vi "UHR-Fleezers Control (host) - 10.8MV_trial2.vi"() -> ()   [LabVIEW 2010] (continued)
        n697 = xnode "Read/Write Control"("FPGA VI Reference In"=w3157, "error in"=w3156, "Invert APD Gate"=w3154, "APD Gate ON Count"=w3153, "APD Gate OFF Count"=w3152, "APD Acq Rate Count"=w3148, "APD Gate Operating Mode"=w3151, "APD 1 AO scale factor"=w3146, "APD 2 AO scale factor"=w3145) -> ("error out"=w3155:errorcluster)  [unwired: 1 out]
      }
      event "GI Frequency, ON count", "Green FB Count", "GI Frequency, OFF count": Value Change {
        n698 = event-data() -> ()  [unwired: 7 out]
        n699 = xnode "Read/Write Control"("FPGA VI Reference In"=w3321, "error in"=w3319, "Green interlace ON count"="GI Frequency, ON count", "Green interlace OFF count"="GI Frequency, OFF count", "Green interlace ON count 2"="GI Frequency, ON count", "Green interlace OFF count 2"="GI Frequency, OFF count", "Green FB Count"="Green FB Count") -> ("error out"=w3320:errorcluster)  [unwired: 1 out]
      }
      event "Number of F/B Scans (AOD)", "Scan Speed (nm/s)", "Scan BD", "Initial delta (MHz)", "Step Size (nm)", "Scan Range (nm)": Value Change {
        w3500 = 123.0  # AOM cal (nm/MHz)
        n700 = event-data() -> ()  [unwired: 7 out]
        n701 = local read "BD 1 Frequency 1 (MHz)"() -> (w3483:dbl)
        n702 = local read "AOM X Cal (nm/MHz)"() -> (w3475:dbl)
        n703 = local read "X RF Frequency Limits (MHz)"() -> (w3487:T16)
        n704 = local read "Y RF Frequency Limits (MHz)"() -> (w3484:T16)
        n705 = local read "BD 2 Frequency 1 (MHz)"() -> (w3489:dbl)
        n706 = Negate(x="Scan Range (nm)") -> (-x=w3453:dbl)
        n707 = Divide(x=w3453, y=w3475) -> (x/y=w3457:dbl)
        n708 = Select(t=w3487, s="Scan BD", f=w3484) -> (s? t:f=w3486:T16)
        n709 = Select(t=w3483, s="Scan BD", f=w3489) -> (s? t:f=w3488:dbl)
        n710 = Unbundle By Name(w3486) -> ("Maximum"=w3495:dbl, "Minimum"=w3494:dbl)
        n711 = Add(x=w3457, y=w3488) -> (x+y=w3492:dbl)
        n712 = Divide(x=w3453, y="Step Size (nm)") -> (x/y=w3472:dbl)
        n713 = Divide(x="Step Size (nm)", y=w3475) -> (x/y=w3481:dbl)
        n714 = Absolute Value(x=w3472) -> (abs(x)=w3456:dbl)
        n715 = Sign(1:w3453) -> (0:w3454:dbl)
        n716 = In Range and Coerce(upper limit=w3495, x=w3492, lower limit=w3494) -> (coerced(x)=w3491:dbl, In Range?=w3493:bool)
        n717 = To Unsigned Quad Integer(1:w3456) -> (0:w3471:u64)
        "Scan steps (AOD)" <- w3471
        n718 = call "IR AOM freq to word.vi"("Frequency In (MHz)"=w3481) -> ("Frequency Word Out (double)"=w3478:dbl)
        n719 = Multiply(x=w3454, y=w3478) -> (x*y=w3455:dbl)
        n720 = Subtract(x=w3492, y=w3491) -> (x-y=w3490:dbl)
        n721 = To Quad Integer(1:w3455) -> (0:w3477:i64)
        "Incr. int (AOD)" <- w3477
        n722 = Subtract(x=w3457, y=w3490) -> (x-y=w3476:dbl)
        "Scan Range (MHz)" <- w3476
        n723 = Select(t=w3457, s=w3493, f=w3476) -> (s? t:f=w3496:dbl)
        n724 = Multiply(x=w3476, y=w3475) -> (x*y=w3474:dbl)
        n725 = Decrement(x=w3471) -> (x-1=w3524:u64)
        n726 = Negate(x=w3474) -> (-x=w3470:dbl)
        n727 = local write "Scan Range (nm)"(w3470) -> ()
        n728 = Divide(x=w3496, y=w3524) -> (x/y=w3480:dbl)
        "Scan Increment (MHz)" <- w3480
        n729 = call "IR AOM freq to word.vi"("Frequency In (MHz)"=w3480) -> ("Frequency Word Out (double)"=w3479:dbl)
        n730 = Divide(x="Step Size (nm)", y="Scan Speed (nm/s)") -> (x/y=w3467:dbl)
        n731 = To Quad Integer(1:w3479) -> ()  [unwired: 1 out]
        n732 = local read "Number Interlace Sets"() -> (w3451:u8)
        n733 = local read "AI Count (ticks)"() -> (w3452:u32)
        n734 = local read "Total Counts (ticks)"() -> (w3450:u32)
        n735 = local read "# Samples/trap"() -> (w3482:u32)
        n736 = Multiply(x=w3452, y=w3451) -> (x*y=w3449:u32)
        n737 = Divide(x=w3450, y=w3449) -> (x/y=w3448:dbl)
        n738 = Select(t=w3483, s="Scan BD", f=w3489) -> (s? t:f=w3521:dbl)
        "Initial freq. (MHz)" <- w3521
        n739 = Add(x=w3496, y=w3521) -> (x+y=→"Final freq. (MHz)":dbl)
        n740 = Divide(x=w3450, y=40000000.0) -> (x/y=w3466:dbl)
        n741 = Divide(x=w3467, y=w3466) -> (x/y=w3465:dbl)
        n742 = To Unsigned Quad Integer(1:w3465) -> (0:w3440:u64)
        n743 = Quotient & Remainder(x=w3440, y=u64 2) -> (x-y*floor(x/y)=w3444:u64)  [unwired: 1 out]
        n744 = Equal?(x=w3444, y=u64 0) -> (x = y?=w3442:bool)
        n745 = Decrement(x=w3440) -> (x-1=w3441:u64)
        n746 = Select(t=w3440, s=w3442, f=w3441) -> (s? t:f=w3439:u64)
        "Cycles/step (AOD)" <- w3439
        n747 = xnode "Read/Write Control"("FPGA VI Reference In"=w3532, "error in"=w3531, "Scan steps"=w3471, "Number of scans"="Number of F/B Scans (AOD)", "Cycles per step"=w3439, "Scan freq.  increment"=w3477, "Scan BD"="Scan BD") -> ("error out"=w3530:errorcluster)  [unwired: 1 out]
        n748 = Multiply(x=w3471, y=w3439) -> (x*y=w3525:u64)
        n749 = Multiply(x=w3525, y=u64 2) -> (x*y=w3447:u64)
        n750 = Multiply(x=w3448, y=w3447) -> (x*y=w3446:dbl)
        "Data points/scan (f/b)" <- w3446
        n751 = Multiply(x=w3446, y="Number of F/B Scans (AOD)") -> (x*y=w3528:dbl)
        "Data points/scans" <- w3528
        n752 = Divide(x=w3528, y=w3482) -> (x/y=→"N sets should be saved":dbl)
        n753 = Multiply(x=w3525, y=w3466) -> (x*y=w3464:dbl)
        "Time/Scan (s) (AOD)" <- w3464
        n754 = Select(t=w3496, s="Scan BD", f=0.0) -> (s? t:f=w3522:dbl)
        n755 = Select(t=0.0, s="Scan BD", f=w3496) -> (s? t:f=w3518:dbl)
        n756 = local read "BD 2 Frequency 2 (MHz)"() -> (w3514:dbl)
        n757 = local read "BD 1 Frequency 2 (MHz)"() -> (w3517:dbl)
        n758 = Add(x=w3518, y=w3489) -> (x+y=w3515:dbl)
        n759 = Add(x=w3483, y=w3522) -> (x+y=w3516:dbl)
        n760 = Multiply(x=w3464, y=2.0) -> (x*y=w3463:dbl)
        n761 = Multiply(x=w3463, y="Number of F/B Scans (AOD)") -> (x*y=w3460:dbl)
        n762 = Divide(x=w3460, y=60.0) -> (x/y=→"Time to Finish All (min)":dbl)
        n763 = Add(x="Trap 2 Bead Size (nm)", y="Trap 1 Bead Size (nm)") -> (x+y=w3504:dbl)
        n764 = local read "Initial delta (MHz)"() -> (w3501:dbl)
        n765 = Divide(x=w3504, y=2.0) -> (x/y=w3498:dbl)
        n766 = Subtract(x=w3515, y=w3514) -> (x-y=w3512:dbl)
        n767 = Subtract(x=w3516, y=w3517) -> (x-y=w3513:dbl)
        n768 = Square(x=w3512) -> (x^2=w3511:dbl)
        n769 = Square(x=w3513) -> (x^2=w3510:dbl)
        n770 = Add(x=w3510, y=w3511) -> (x+y=w3509:dbl)
        n771 = Square Root(x=w3509) -> (sqrt(x)=w3508:dbl)
        "Final delta (MHz)" <- w3508
        n772 = Multiply(x=w3500, y=w3508) -> (x*y=w3507:dbl)
        n773 = Multiply(x=w3501, y=w3500) -> (x*y=w3499:dbl)
        n774 = Subtract(x=w3499, y=w3498) -> (x-y=→"Initial sep (nm)":dbl)
        n775 = Subtract(x=w3507, y=w3498) -> (x-y=→"Final sep (nm)":dbl)
      }
      event "Raster Scanning...": Value Change {
        n776 = event-data() -> ("NewVal"=w3669:bool)  [unwired: 6 out]
        n777 = case shown="True" w3669 {
          frame False {
          }
          frame True {
            n778 = property on="BD 1 Frequency 1 (MHz)" class="DigNum (strict)"("Val(Sgnl)"=65.0 ("Value (Signaling)")) -> ()  [unwired: 2 in, 2 out]
          }
        }
      }
      event "Freq or Amp switch first", "Swap F1 and F2", "Freq switch delay", "Amp switch delay": Value Change {
        n779 = event-data() -> ()  [unwired: 7 out]
        n780 = local read "Freq or Amp switch first"() -> (w3671:bool)
        n781 = local read "Amp switch delay"() -> (w3672:u16)
        n782 = local read "Freq switch delay"() -> (w3674:u16)
        n783 = local read "Swap F1 and F2"() -> (w3673:bool)
        n784 = xnode "Read/Write Control"("FPGA VI Reference In"=w3677, "error in"=w3676, "Freq switch delay"=w3674, "Swap F1 and F2"=w3673, "Amp switch delay"=w3672, "Freq or Amp switch first"=w3671) -> ("error out"=w3675:errorcluster)  [unwired: 1 out]
      }
      event "Scan steps (MCL)", "Number of scans (MCL)", "Scan Range (V)\n(of steps)", "2D or 1D Scan", "N APD Samp/step", "Fast Scan Dir", "Continuous MCL Scanning", "Scan lines (y)": Value Change {
        w3778 = 32767.0 ("y")
        n785 = event-data() -> ()  [unwired: 7 out]
        n786 = Select(t="Scan lines (y)", s="2D or 1D Scan", f="Number of scans (MCL)") -> (s? t:f=w3783:u64)
        n787 = Decrement(x="Scan steps (MCL)") -> (x-1=w3799:u64)
        n788 = Divide(x="Scan Range (V)\n(of steps)", y=w3799) -> (x/y=w3798:dbl)
        "Desired Scan Incr (V)" <- w3798
        n789 = local read "APD Integration Time (s)"() -> (w3791:dbl)
        n790 = Multiply(x=w3798, y=w3778) -> (x*y=w3807:dbl)
        n791 = Divide(x=w3807, y=10.0) -> (x/y=w3797:dbl)
        "Desired incr (int)" <- w3797
        n792 = local read "Update Count (MCL)"() -> (w3803:u32)
        n793 = Round Toward -Infinity(1:w3797) -> (0:w3806:dbl)
        n794 = To Word Integer(number=w3806) -> (16bit integer=w3781:i16)
        "Actual Incr. int (MCL)" <- w3781
        n795 = Multiply(x=w3791, y=40000000.0) -> (x*y=w3804:dbl)
        n796 = Divide(x=w3804, y=w3803) -> (x/y=w3802:dbl)
        n797 = Multiply(x=i16 10, y=w3781) -> (x*y=w3779:i16)
        n798 = Multiply(x="N APD Samp/step", y=w3802) -> (x*y=w3801:dbl)
        "Cycles/step (MCL)" <- w3801
        n799 = Divide(x=w3779, y=w3778) -> (x/y=→"Actual MCL Inc (V)":dbl)
        n800 = Multiply(x="N APD Samp/step", y="Scan steps (MCL)") -> (x*y=w3793:dbl)
        n801 = local read "APD Samples/FIFO Acq."() -> (w3790:dbl)
        n802 = Multiply(x=w3793, y=u64 2) -> (x*y=w3792:dbl)
        "Data points/scan (f+b)" <- w3792
        n803 = Multiply(x=w3792, y=w3783) -> (x*y=w3810:dbl)
        "Data points/scans (MCL)" <- w3810
        n804 = Multiply(x=w3791, y=w3792) -> (x*y=w3784:dbl)
        "Time/f+b scan (s) (MCL)" <- w3784
        n805 = Divide(x=w3810, y=w3790) -> (x/y=→"N sets should be saved (MCL)":dbl)
        n806 = Multiply(x=w3784, y=w3783) -> (x*y=→"Total Time (s)":dbl)
        n807 = Not(x="Fast Scan Dir") -> (.not. x?=w3788:bool)
        n808 = xnode "Read/Write Control"("FPGA VI Reference In"=w3814, "error in"=w3813, "Scan steps (MCL)"="Scan steps (MCL)", "Number of scans (MCL)"=w3783, "Cycles per step (MCL)"=w3801, "Scan freq.  increment (MCL)"=w3781, "1D or 2D Scan?"="2D or 1D Scan", "MCL Scan Axis"=w3788, "Cont. Scan (MCL)"="Continuous MCL Scanning") -> ("error out"=w3812:errorcluster)  [unwired: 1 out]
      }
      event "Read Cal": Value Change {
        w3988 = 1000.0 ("y")
        n809 = event-data() -> ()  [unwired: 7 out]
        n810 = local read "Save file name"() -> (w4013:path)
        n811 = local write "Read Cal"(FALSE ("Read Cal")) -> ()
        n812 = Strip Path(path=w4013) -> (stripped path=w4012:path)  [unwired: 1 out]
        n813 = Path To String(path=w4012) -> (string=w4011:string)
        n814 = Concatenate Strings(w4011, "\\current.cal" ("string")) -> (w4009:string)
        n815 = String To Path(string=w4009) -> (path=w4008:path)
        n816 = Open/Create/Replace File(file path (use dialog)=w4008, operation (0:open)=T25."open", access (0:read/write)=enum16{"read/write", "read-only", "write-only"}."read-only") -> (refnum out=w4016:refnum<file>, error out=w4002:errorcluster)  [unwired: 1 in, 3 out]
        n817 = Deny Access(4:w4002, 7:w4016) -> (0:w4001:errorcluster, 3:w4007:refnum<file>)  [unwired: 1 out]
        n818 = Read from Binary File(5:0.0, 8:w4001, 9:T31."big-endian, network order" ("byte order (0:big-endian, network order)"), 10:-1 ("count (1)"), 11:w4007) -> (0:w4000:errorcluster, 2:w3998:dbl[], 3:w4003:refnum<file>)  [unwired: 2 out]
        n819 = Array To Cluster(array=w3998) -> (cluster=w3997:T33)
        n820 = Unbundle(w3997) -> ("[0]"=w3996:dbl, "[1]"=w3995:dbl, "[2]"=w3994:dbl, "[3]"=w3993:dbl, "[4]"=w3992:dbl, "[5]"=w3991:dbl)
        n821 = Close File(refnum=w4003, error in=w4000) -> (error out=→"Read cal error":errorcluster)  [unwired: 1 out]
        n822 = Multiply(x=w3991, y=w3988) -> (x*y=w3989:dbl)
        n823 = local write "T2 kappa_x (pN/nm)"(w3993) -> ()
        n824 = local write "T1 kappa_x (pN/nm)"(w3994) -> ()
        n825 = local write "T1 alpha_x (nm/V)"(w3996) -> ()
        n826 = local write "T2 alpha_x (nm/V)"(w3995) -> ()
        n827 = Multiply(x=w3992, y=w3988) -> (x*y=w3990:dbl)
        n828 = local write "T1 offset_x (mV)"(w3990) -> ()
        n829 = local write "T2 offset_x (mV)"(w3989) -> ()
      }
      event "Abort MCL Scan": Value Change {
        n830 = event-data() -> ()  [unwired: 7 out]
        n831 = local write "MCL Scanning"(FALSE ("MCL Scanning")) -> ()
        n832 = xnode "Read/Write Control"("FPGA VI Reference In"=w4021, "error in"=w4020, "Abort scan (MCL)"="Abort MCL Scan") -> ("error out"=w4019:errorcluster)  [unwired: 1 out]
      }
      event "Update Count (MCL)": Value Change {
        n833 = event-data() -> ()  [unwired: 7 out]
        n834 = xnode "Read/Write Control"("FPGA VI Reference In"=w4063, "error in"=w4062, "MCL count"="Update Count (MCL)") -> ("error out"=w4061:errorcluster)  [unwired: 1 out]
      }
      event "Phase adjust (MCL)", "+ phase (MCL)", "- phase (MCL)": Value Change {
        n835 = event-data() -> ()  [unwired: 7 out]
        n836 = Negate(x="Phase adjust (MCL)") -> (-x=w4109:i16)
        n837 = Select(t=w4109, s="- phase (MCL)", f="Phase adjust (MCL)") -> (s? t:f=w4107:i16)
        n838 = Or(x="- phase (MCL)", y="+ phase (MCL)") -> (x .or. y?=w4102:bool)
        n839 = xnode "Read/Write Control"("FPGA VI Reference In"=w4111, "error in"=w4110, "Phase count adjustment (MCL)"=w4107) -> ("FPGA VI Reference Out"=w4103:T19, "error out"=w4104:errorcluster)
        n840 = xnode "Read/Write Control"("FPGA VI Reference In"=w4103, "error in"=w4104, "+ phase (MCL)"=w4102) -> ("error out"=w4101:errorcluster)  [unwired: 1 out]
      }
      event "Abort AOD Scan": Value Change {
        n841 = event-data() -> ()  [unwired: 7 out]
        n842 = xnode "Read/Write Control"("FPGA VI Reference In"=w4190, "error in"=w4189, "Abort scan"="Abort AOD Scan") -> ("error out"=w4188:errorcluster)  [unwired: 1 out]
      }
      event "Continuous AOD Scanning": Value Change {
        n843 = event-data() -> ()  [unwired: 7 out]
        n844 = xnode "Read/Write Control"("FPGA VI Reference In"=w4232, "error in"=w4231, "Cont. Scan"="Continuous AOD Scanning") -> ("error out"=w4230:errorcluster)  [unwired: 1 out]
      }
      event "Index": Value Change {
        n845 = event-data() -> ()  [unwired: 7 out]
        n846 = call "Create new save file.vi"("Insert"="", "Ext"=".dat" ("string"), "Index In"="Index") -> ("Path Out"=→"Save file name":path, "Index Out"=w4271:dbl)
        "Save index" <- w4271
        n847 = local write "Index"(w4271) -> ()
      }
      event "AO1", "AO2": Value Change {
        w4286 = 10.0 ("y")
        w4285 = 32767.0 ("y")
        n848 = event-data() -> ()  [unwired: 7 out]
        n849 = local read "AO2"() -> (w4284:dbl)
        n850 = local read "AO1"() -> (w4281:dbl)
        n851 = Multiply(x=w4281, y=w4285) -> (x*y=w4280:dbl)
        n852 = Multiply(x=w4284, y=w4285) -> (x*y=w4283:dbl)
        n853 = Divide(x=w4280, y=w4286) -> (x/y=w4279:dbl)
        n854 = Divide(x=w4283, y=w4286) -> (x/y=w4282:dbl)
        n855 = To Word Integer(number=w4279) -> (16bit integer=w4287:i16)
        n856 = To Word Integer(number=w4282) -> (16bit integer=w4288:i16)
        n857 = xnode "Read/Write Control"("FPGA VI Reference In"=w4278, "error in"=w4277, "AO1"=w4287, "AO2"=w4288) -> ("error out"=w4276:errorcluster)  [unwired: 1 out]
      }
      event "Inject Bottom": Value Change {
        n858 = event-data() -> ()  [unwired: 7 out]
        n859 = disable-structure shown="Enabled" {
          disable-tunnel: "Inject Bottom" -> [w4347 w4387]
          frame Disabled {
            n860 = local read "Chemyx Syringe Pump Serial Port"() -> (w4348:refnum<visa-resource-name>)
            n861 = local read "Pump write delay (ms)"() -> (w4349:dbl)
            n862 = case shown="True" w4347 {
              tunnel: w4349 -> [w4355 w4369]
              tunnel: w4348 -> [w4352 w4368]
              frame False {
                n863 = flat-sequence {
                  tunnel: w4352 -> [w4356]
                  tunnel: [w4356] -> w4353
                  tunnel: w4355 -> [_]
                  tunnel: [w4359] -> w4354
                  tunnel: w4353 -> [w4359]
                  tunnel: w4354 -> [w4360]
                  tunnel: [w4360] -> w4350
                  tunnel: [w4362] -> w4351
                  tunnel: w4350 -> [w4362]
                  tunnel: w4351 -> [w4364]
                  frame #0 {
                    n864 = call "Write to pump.vi"("string"="enter pump1", "VISA resource name"=w4356) -> ()  [unwired: 1 out]
                  }
                  frame #1 {
                    n865 = Wait (ms)(milliseconds to wait="Pump pause delay (ms)") -> ()  [unwired: 1 out]
                  }
                  frame #2 {
                    n866 = call "Write to pump.vi"("string"="stop", "VISA resource name"=w4360) -> ()  [unwired: 1 out]
                  }
                  frame #3 {
                    n867 = Wait (ms)(milliseconds to wait=u32 500) -> ()  [unwired: 1 out]
                  }
                  frame #4 {
                    n868 = call "Write to pump.vi"("string"="stop", "VISA resource name"=w4364) -> ()  [unwired: 1 out]
                  }
                }
              }
              frame True {
                n869 = flat-sequence {
                  tunnel: w4368 -> [w4378]
                  tunnel: w4369 -> [w4373]
                  tunnel: w4369 -> [w4380]
                  tunnel: w4368 -> [w4381]
                  tunnel: [w4381] -> w4366
                  tunnel: [w4383] -> w4367
                  tunnel: w4366 -> [w4383]
                  tunnel: w4367 -> [w4385]
                  frame #0 {
                    n870 = local read "All Pump Parameters"() -> (w4372:T5)
                    n871 = Unbundle By Name(w4372) -> ("Pump 1"=w4379:T34)
                    n872 = call "Set pump parameters.vi"("Pump write delay (ms)"=w4373, "Volume (uL)"="Ch 2 Inject Volume (uL)", "Rate (uL/h)"="Ch 1 Inject Rate (ul/h)", "Units"=4.0, "Pump #"=1.0, "Pump Parameters In"=w4379, "VISA resource name"=w4378) -> ("Pump Parameters Out"=w4371:T34)  [unwired: 3 in]
                    n873 = Bundle By Name(cluster=w4372, "Pump 1"=w4371) -> (w4370:T5)
                    n874 = local write "All Pump Parameters"(w4370) -> ()
                  }
                  frame #1 {
                    n875 = Wait (ms)(milliseconds to wait=w4380) -> ()  [unwired: 1 out]
                  }
                  frame #2 {
                    n876 = call "Write to pump.vi"("string"="start", "VISA resource name"=w4381) -> ()  [unwired: 1 out]
                  }
                  frame #3 {
                    n877 = Wait (ms)(milliseconds to wait=u32 500) -> ()  [unwired: 1 out]
                  }
                  frame #4 {
                    n878 = call "Write to pump.vi"("string"="start", "VISA resource name"=w4385) -> ()  [unwired: 1 out]
                  }
                }
              }
            }
          }
          frame Enabled {
            n879 = call "hamilton_controller.vi"("Open?"=w4387, "valve"=enum16{"A", "B", "C", "D", "ALL"}."B", "action"=T22."MOVE VALVE") -> ()  [unwired: 8 in, 1 out]
          }
        }
      }
      event "Inject Top": Value Change {
        n880 = event-data() -> ()  [unwired: 7 out]
        n881 = disable-structure shown="Disabled" {
          disable-tunnel: "Inject Top" -> [_ w4431]
          frame Disabled {
            n882 = local read "Pump write delay (ms)"() -> (w4392:dbl)
            n883 = case shown="False" w4393 {
              tunnel: w4392 -> [w4399 w4413]
              tunnel: "Chemyx Syringe Pump Serial Port" -> [w4396 w4412]
              frame False {
                n884 = flat-sequence {
                  tunnel: w4396 -> [w4400]
                  tunnel: [w4400] -> w4397
                  tunnel: w4399 -> [_]
                  tunnel: [w4403] -> w4398
                  tunnel: w4397 -> [w4403]
                  tunnel: w4398 -> [w4404]
                  tunnel: [w4404] -> w4394
                  tunnel: [w4406] -> w4395
                  tunnel: w4394 -> [w4406]
                  tunnel: w4395 -> [w4408]
                  frame #0 {
                    n885 = call "Write to pump.vi"("string"="enter pump3", "VISA resource name"=w4400) -> ()  [unwired: 1 out]
                  }
                  frame #1 {
                    n886 = local read "Pump pause delay (ms)"() -> (w4402:u32)
                    n887 = Wait (ms)(milliseconds to wait=w4402) -> ()  [unwired: 1 out]
                  }
                  frame #2 {
                    n888 = call "Write to pump.vi"("string"="stop", "VISA resource name"=w4404) -> ()  [unwired: 1 out]
                  }
                  frame #3 {
                    n889 = Wait (ms)(milliseconds to wait=u32 0) -> ()  [unwired: 1 out]
                  }
                  frame #4 {
                    n890 = call "Write to pump.vi"("string"="stop", "VISA resource name"=w4408) -> ()  [unwired: 1 out]
                  }
                }
              }
              frame True {
                n891 = flat-sequence {
                  tunnel: w4412 -> [w4422]
                  tunnel: w4413 -> [w4417]
                  tunnel: w4413 -> [w4424]
                  tunnel: w4412 -> [w4425]
                  tunnel: [w4425] -> w4410
                  tunnel: [w4428] -> w4411
                  tunnel: w4410 -> [w4428]
                  tunnel: w4411 -> [w4429]
                  frame #0 {
                    n892 = local read "All Pump Parameters"() -> (w4416:T5)
                    n893 = Unbundle By Name(w4416) -> ("Pump 3"=w4423:T34)
                    n894 = call "Set pump parameters.vi"("Pump write delay (ms)"=w4417, "Volume (uL)"="Ch 3 Inject Volume (uL)", "Rate (uL/h)"="Ch 3 Inject Rate (ul/h)", "Units"=4.0, "Pump #"=3.0, "Pump Parameters In"=w4423, "VISA resource name"=w4422) -> ("Pump Parameters Out"=w4415:T34)  [unwired: 3 in]
                    n895 = Bundle By Name(cluster=w4416, "Pump 3"=w4415) -> (w4414:T5)
                    n896 = local write "All Pump Parameters"(w4414) -> ()
                  }
                  frame #1 {
                    n897 = Wait (ms)(milliseconds to wait=w4424) -> ()  [unwired: 1 out]
                  }
                  frame #2 {
                    n898 = call "Write to pump.vi"("string"="start", "VISA resource name"=w4425) -> ()  [unwired: 1 out]
                  }
                  frame #3 {
                    n899 = Wait (ms)(milliseconds to wait=u32 500) -> ()  [unwired: 1 out]
                  }
                  frame #4 {
                    n900 = call "Write to pump.vi"("string"="start", "VISA resource name"=w4429) -> ()  [unwired: 1 out]
                  }
                }
              }
            }
          }
          frame Enabled {
            n901 = call "hamilton_controller.vi"("Open?"=w4431, "valve"=enum16{"A", "B", "C", "D", "ALL"}."A", "action"=T22."MOVE VALVE") -> ()  [unwired: 8 in, 1 out]
          }
        }
      }
      event "Inject Valve B": Value Change {
        n902 = event-data() -> ()  [unwired: 7 out]
        n903 = disable-structure shown="Enabled" {
          disable-tunnel: "Inject Valve B" -> [w4435 w4455]
          frame Disabled {
            n904 = local read "Pump write delay (ms)"() -> (w4437:dbl)
            n905 = flat-sequence {
              tunnel: w4436 -> [w4450]
              tunnel: w4437 -> [w4446]
              tunnel: w4435 -> [_]
              tunnel: w4437 -> [w4452]
              tunnel: w4436 -> [w4453]
              frame #0 {
                n906 = local read "All Pump Parameters"() -> (w4445:T5)
                n907 = Multiply(x=60.0, y="Flush Center Ch Rate (ul/m)") -> (x*y=w4442:dbl)
                n908 = Unbundle By Name(w4445) -> ("Pump 2"=w4451:T34)
                n909 = call "Set pump parameters.vi"("Pump write delay (ms)"=w4446, "Volume (uL)"="Flush Center Ch Volume (uL)", "Rate (uL/h)"=w4442, "Units"=3.0, "Pump #"=2.0, "Pump Parameters In"=w4451, "VISA resource name"=w4450) -> ("Pump Parameters Out"=w4444:T34)  [unwired: 3 in]
                n910 = Bundle By Name(cluster=w4445, "Pump 2"=w4444) -> (w4443:T5)
                n911 = local write "All Pump Parameters"(w4443) -> ()
                n912 = Add(x="Flush Center Ch Volume (uL)", y="Total Volume\nFlushed (uL)") -> (x+y=w4439:dbl)
                n913 = local write "Total Volume\nFlushed (uL)"(w4439) -> ()
              }
              frame #1 {
                n914 = Wait (ms)(milliseconds to wait=w4452) -> ()  [unwired: 1 out]
              }
              frame #2 {
                n915 = call "Write to pump.vi"("string"="start", "VISA resource name"=w4453) -> ()  [unwired: 1 out]
              }
            }
            n916 = local read "Chemyx Syringe Pump Serial Port"() -> (w4436:refnum<visa-resource-name>)
          }
          frame Enabled {
            n917 = call "hamilton_controller.vi"("Open?"=w4455, "valve"=enum16{"A", "B", "C", "D", "ALL"}."B", "action"=T22."MOVE VALVE") -> ()  [unwired: 8 in, 1 out]
          }
        }
      }
      event "Sample Channel Flow": Value Change {
        n918 = event-data() -> ()  [unwired: 7 out]
        n919 = call "hamilton_controller.vi"("Open?"="Sample Channel Flow", "valve"=enum16{"A", "B", "C", "D", "ALL"}."C", "action"=T22."MOVE VALVE") -> ()  [unwired: 8 in, 1 out]
      }
      event "Flip Green Filter": Value Change {
        n920 = event-data() -> ()  [unwired: 7 out]
        n921 = Not(x="Flip Green Filter") -> (.not. x?=w4461:bool)
        n922 = local write "Flip Green Filter"(w4461) -> ()
        n923 = flat-sequence {
          tunnel: w4469 -> [w4474]
          tunnel: w4468 -> [w4473]
          tunnel: [w4471] -> w4466
          tunnel: [w4470] -> w4465
          tunnel: [w4514] -> w4464
          tunnel: w4466 -> [w4514]
          tunnel: [w4513] -> w4463
          tunnel: w4465 -> [w4513]
          tunnel: w4464 -> [w4518]
          tunnel: w4463 -> [w4517]
          tunnel: [w4516] -> w4467
          frame #0 {
            n924 = xnode "Read/Write Control"("FPGA VI Reference In"=w4474, "error in"=w4473, "Green Filter Flipper"=TRUE) -> ("FPGA VI Reference Out"=w4471:T19, "error out"=w4470:errorcluster)
          }
          frame #1 {
            n925 = Wait (ms)(milliseconds to wait=u32 100) -> ()  [unwired: 1 out]
          }
          frame #2 {
            n926 = xnode "Read/Write Control"("FPGA VI Reference In"=w4518, "error in"=w4517, "Green Filter Flipper"=FALSE) -> ("error out"=w4516:errorcluster)  [unwired: 1 out]
          }
        }
      }
      event "Pump 1 contents", "Pump 3 contents": Value Change {
        n927 = event-data() -> ()  [unwired: 7 out]
        n928 = local read "Pump 1 contents"() -> (→"Pump 1 cont disp":string)
        n929 = local read "Pump 3 contents"() -> (→"Pump 3 cont disp":string)
      }
      event "Reset Trap Pos. FB": Value Change {
        n930 = event-data() -> ()  [unwired: 7 out]
        n931 = xnode "Read/Write Control"("FPGA VI Reference In"=w4562, "error in"=w4561, "Trap Pos. FB Reset"="Reset Trap Pos. FB") -> ()  [unwired: 2 out]
      }
      event "Trap Pos. FB ON": Value Change {
        n932 = event-data() -> ()  [unwired: 7 out]
        n933 = xnode "Read/Write Control"("FPGA VI Reference In"=w4603, "error in"=w4602, "Force feedback"="Trap Pos. FB ON") -> ()  [unwired: 2 out]
      }
      event "Trap Pos. FB Range", "Trap Pos. FB Gains", "Trap Pos. FB Mult Factor", "Trap Pos. FB Offset Factor", "Trap Pos FB Negate Action", "Trap Pos FB Monitor\nT1 or T2": Value Change {
        n934 = event-data() -> ()  [unwired: 7 out]
        n935 = xnode "Read/Write Control"("FPGA VI Reference In"=w4650, "error in"=w4649, "Trap Pos. FB Range"="Trap Pos. FB Range", "Trap Pos. FB Gains"="Trap Pos. FB Gains", "Trap Pos. FB Mult Factor"="Trap Pos. FB Mult Factor", "Trap Pos. FB Offset Factor"="Trap Pos. FB Offset Factor", "Trap Pos FB Negate Action"="Trap Pos FB Negate Action", "Trap Pos FB Monitor T1 or T2"="Trap Pos FB Monitor\nT1 or T2", "AI1 X Scale"="Trap Pos. AI1 X Pre-scale") -> ()  [unwired: 2 out]
      }
      event "Trap Pos FB SP": Value Change {
        n936 = event-data() -> ()  [unwired: 7 out]
        n937 = xnode "Read/Write Control"("FPGA VI Reference In"=w4838, "error in"=w4837, "Trap Pos. FB SP"="Trap Pos FB SP") -> ()  [unwired: 2 out]
      }
      event "Set SP to Reading": Value Change {
        n938 = event-data() -> ()  [unwired: 7 out]
        n939 = local read "Trap Pos FB Monitor\nT1 or T2"() -> (w4891:bool)
        n940 = local read "Trap X AI1 (DMA)"() -> (w4894:T13)
        n941 = local read "Trap X (AI1)"() -> (w4897:T10)
        n942 = Unbundle By Name(w4897) -> ("Trap 1"=w4896:fxp<+/-,16,1>, "Trap 2"=w4895:fxp<+/-,16,1>)
        n943 = Unbundle By Name(w4894) -> ("Set 1"=w4893:fxp<+/-,16,1>, "Set 2"=w4892:fxp<+/-,16,1>)
        n944 = Select(t=w4896, s=w4891, f=w4895) -> (s? t:f=w4890:fxp<+/-,16,1>)
        n945 = Select(t=w4893, s=w4891, f=w4892) -> (s? t:f=w4889:fxp<+/-,16,1>)
        n946 = Not(x="Set SP Using...") -> (.not. x?=w4884:bool)
        n947 = Select(t=w4890, s=w4884, f=w4889) -> (s? t:f=w4885:fxp<+/-,16,1>)
        n948 = xnode "Read/Write Control"("FPGA VI Reference In"=w4887, "error in"=w4886, "Trap Pos. FB SP"=w4885) -> ()  [unwired: 2 out]
        n949 = local write "Trap Pos FB SP"(w4885) -> ()
      }
      event "Trap Pos. FB Out Scale 2^n": Value Change {
        n950 = event-data() -> ()  [unwired: 7 out]
        n951 = Scale By Power Of 2(n="Trap Pos. FB Out Scale 2^n", x=ext 1.0) -> (x*2^n=w4944:ext)
        n952 = property on="Trap Pos. FB Mult Factor" class="DigNum (strict)"("Val(Sgnl)"=w4944) -> ()  [unwired: 2 in, 2 out]
      }
      event "Trap Pos FB Int Count": Value Change {
        n953 = event-data() -> ()  [unwired: 7 out]
        n954 = xnode "Read/Write Control"("FPGA VI Reference In"=w4949, "error in"=w4948, "Trap Pos FB Int Count"="Trap Pos FB Int Count") -> ()  [unwired: 2 out]
      }
    }
    "error out 2" <- w1274
    n955 = node-c288() -> ()  [unwired: 1 in, 1 out]
  }
  n956 = timed-loop "Run Scripts, including: stage motion" {
    timing: w69 -> [_]
    timing-out: [_] -> w68
    tunnel: w24 -> [_]
    stop <- w4988 stop-if-true
    n957 = node-c288() -> ()  [unwired: 1 in, 1 out]
    n958 = event shown="[2] \"Cal/Data Acq. Spot\": Value Change" {
      selector: _ -> [_ _ _ _ _ _ _ _ _ _ _ _]
      dyn-events: _ -> [_ _ _ _ _ _ _ _ _ _ _ _]
      timeout: 50 -> [_ _ _ _ _ _ _ _ _ _ _ _]
      tunnel: ["Move Cap. 1 (DNA Top)" _ "Cal/Data Acq. Spot" "Dump Beads" "Dip for Protein" _ "Got ADig bead" "Got DNA bead" "Take Stepping Data" _ "Take Detection Laser\nImage" _] -> _
      tunnel: [_ _ _ _ _ _ _ _ _ _ _ w5192] -> w4988
      event "Move Cap. 1 (DNA Top)": Value Change {
        n959 = event-data() -> ()  [unwired: 1 in, 5 out]
        n960 = local write "Move Cap. 1 (DNA Top)"(FALSE ("Move Cap. 1 (DNA Right)")) -> ()
        n961 = flat-sequence {
          tunnel: "Cap 1 Samp Flow ON" -> [w4994]
          frame #0 {
            n962 = local write "Stage Moving"(FALSE ("Stage Moving")) -> ()
            n963 = case "stop flow" shown="True" w4994 {
              frame False {
              }
              frame True {
                n964 = call "hamilton_controller.vi"("Open?"=FALSE, "valve"=enum16{"A", "B", "C", "D", "ALL"}."C", "action"=T22."MOVE VALVE") -> ()  [unwired: 8 in, 1 out]
              }
            }
            n965 = case shown="True" TRUE {
              tunnel: "Cap 1 T ON" -> [w5003 w5004]
              frame False {
                n966 = property on="Trap 1 (ON/OFF)" class="Bool (strict)"("Val(Sgnl)"=w5003) -> ()  [unwired: 2 in, 2 out]
              }
              frame True {
                n967 = property on="Trap 2 (ON/OFF)" class="Bool (strict)"("Val(Sgnl)"=w5004) -> ()  [unwired: 2 in, 2 out]
              }
            }
            n968 = call <vilib>:"Beep.vi"() -> ()  [unwired: 3 in, 9 out]
            n969 = case shown="True" "Cap 1 Flow ON" {
              frame False {
              }
              frame True {
                n970 = property on="Inject Top" class="Bool (strict)"("Val(Sgnl)"=TRUE ("Value (Signaling)")) -> ()  [unwired: 2 in, 2 out]
              }
            }
          }
        }
      }
      event Timeout {
        n971 = event-data() -> ()  [unwired: 1 in, 2 out]
      }
      event "Cal/Data Acq. Spot": Value Change {
        # "wait for calibration file\nto be written"
        # "signal save cal true\nthis tells the data \nacquisition loop to\nstart sending the data\nto a calibration file"
        # "separate traps to\nthe desired trap delta"
        # "move stage to data acquisition spot"
        # "CHANGE FISH FOR TETHER BACK\nTO TRUE VALUE HERE."
        n972 = event-data() -> ()  [unwired: 1 in, 5 out]
        n973 = local write "Cal/Data Acq. Spot"(FALSE ("Cal/Data Acq. Spot")) -> ()
        n974 = flat-sequence {
          tunnel: ["Cal @ (MHz)"] -> w5005
          tunnel: w5005 -> [w5015]
          tunnel: w5005 -> [w5036]
          frame #0 {
            n975 = property on="Trap Delta (MHz)" class="DigNum (strict)"("Val(Sgnl)"="Cal @ (MHz)") -> ()  [unwired: 2 in, 2 out]
            n976 = call <vilib>:"Beep.vi"() -> ()  [unwired: 3 in, 9 out]
          }
          frame #1 {
            n977 = Wait (ms)(milliseconds to wait=u32 100) -> ()  [unwired: 1 out]
          }
          frame #2 {
            n978 = property on="Save Calibration" class="Bool (strict)"("Val(Sgnl)"=TRUE ("Value (Signaling)")) -> ()  [unwired: 2 in, 2 out]
          }
          frame #3 {
            n979 = Wait (ms)(milliseconds to wait=u32 4000) -> ()  [unwired: 1 out]
          }
          frame #4 {
            n980 = while {
              stop <- w5012 stop-if-true
              n981 = local read "Saving..."() -> (w5013:bool)
              n982 = Wait (ms)(milliseconds to wait=u32 100) -> ()  [unwired: 1 out]
              n983 = Not(x=w5013) -> (.not. x?=w5012:bool)
            }
          }
          frame #5 {
            n984 = case shown="True" "W/ Offset 1" {
              tunnel: w5015 -> [_ w5017]
              frame False {
              }
              frame True {
                n985 = stacked-sequence {
                  tunnel: w5017 -> [_ _ _ _ _ _ _ w5034]
                  frame #0 {
                    n986 = Replace Array Subset(array=u32[] [0] ("Index Values"), new element="Offset 1 Set", index=0) -> (w5018:u32[])
                    n987 = property on="Saved AOD Raster Scan Parameter Sets" class="Arr (strict)"("Index Values"=w5018) -> ()  [unwired: 2 in, 2 out]
                    n988 = property on="Trap Delta (MHz)" class="DigNum (strict)"("Val(Sgnl)"="Offset 1 Start (MHz)") -> ()  [unwired: 2 in, 2 out]
                  }
                  frame #1 {
                    n989 = Wait (ms)(milliseconds to wait=u32 200) -> ()  [unwired: 1 out]
                  }
                  frame #2 {
                    n990 = property on="Load parameters" class="Bool (strict)"("Val(Sgnl)"=TRUE ("Value (Signaling)")) -> ()  [unwired: 2 in, 2 out]
                  }
                  frame #3 {
                    n991 = Wait (ms)(milliseconds to wait=u32 200) -> ()  [unwired: 1 out]
                  }
                  frame #4 {
                    n992 = property on="Trap Raster Scan" class="Bool (strict)"("Val(Sgnl)"=TRUE ("Value (Signaling)")) -> ()  [unwired: 2 in, 2 out]
                  }
                  frame #5 {
                    n993 = Wait (ms)(milliseconds to wait=u32 2000) -> ()  [unwired: 1 out]
                  }
                  frame #6 {
                    n994 = while {
                      stop <- w5031 stop-if-true
                      n995 = local read "Raster Scanning..."() -> (w5033:bool)
                      n996 = local read "Saving..."() -> (w5029:bool)
                      n997 = Wait (ms)(milliseconds to wait=u32 100) -> ()  [unwired: 1 out]
                      n998 = Not(x=w5029) -> (.not. x?=w5028:bool)
                      n999 = Not(x=w5033) -> (.not. x?=w5030:bool)
                      n1000 = And(x=w5030, y=w5028) -> (x .and. y?=w5031:bool)
                    }
                  }
                  frame #7 {
                    n1001 = property on="Trap Delta (MHz)" class="DigNum (strict)"("Val(Sgnl)"=w5034) -> ()  [unwired: 2 in, 2 out]
                  }
                }
              }
            }
          }
          frame #6 {
            n1002 = local read "Save ave N"() -> (w5035:dbl)
            n1003 = case shown="True" "W/ Offset 2" {
              tunnel: w5036 -> [_ w5042]
              tunnel: w5035 -> [_ w5041]
              frame False {
                n1004 = Multiply(x="Cal read wait (s)", y=u32 1000 ("milliseconds to wait")) -> (x*y=w5039:u32)
                n1005 = Wait (ms)(milliseconds to wait=w5039) -> ()  [unwired: 1 out]
              }
              frame True {
                n1006 = stacked-sequence {
                  tunnel: w5042 -> [_ _ _ _ _ _ _ _ _ w5063 _ _]
                  tunnel: w5041 -> [_ _ _ _ _ _ _ _ _ w5061 _ _]
                  frame #0 {
                    n1007 = property on="Save ave N" class="DigNum (strict)"("Val(Sgnl)"=1.0 ("Value (Signaling)")) -> ()  [unwired: 2 in, 2 out]
                  }
                  frame #1 {
                    n1008 = Wait (ms)(milliseconds to wait=u32 500) -> ()  [unwired: 1 out]
                  }
                  frame #2 {
                    n1009 = property on="Trap Delta (MHz)" class="DigNum (strict)"("Val(Sgnl)"="Offset 2 Start (MHz)") -> ()  [unwired: 2 in, 2 out]
                    n1010 = Replace Array Subset(array=u32[] [0] ("Index Values"), new element="Offset 2 Set", index=0) -> (w5047:u32[])
                    n1011 = property on="Saved AOD Raster Scan Parameter Sets" class="Arr (strict)"("Index Values"=w5047) -> ()  [unwired: 2 in, 2 out]
                  }
                  frame #3 {
                    n1012 = Wait (ms)(milliseconds to wait=u32 500) -> ()  [unwired: 1 out]
                  }
                  frame #4 {
                    n1013 = property on="Load parameters" class="Bool (strict)"("Val(Sgnl)"=TRUE ("Value (Signaling)")) -> ()  [unwired: 2 in, 2 out]
                  }
                  frame #5 {
                    n1014 = Wait (ms)(milliseconds to wait=u32 500) -> ()  [unwired: 1 out]
                  }
                  frame #6 {
                    n1015 = property on="Trap Raster Scan" class="Bool (strict)"("Val(Sgnl)"=TRUE ("Value (Signaling)")) -> ()  [unwired: 2 in, 2 out]
                  }
                  frame #7 {
                    n1016 = Wait (ms)(milliseconds to wait=u32 2000) -> ()  [unwired: 1 out]
                  }
                  frame #8 {
                    n1017 = while {
                      stop <- w5056 stop-if-true
                      n1018 = local read "Raster Scanning..."() -> (w5059:bool)
                      n1019 = local read "Saving..."() -> (w5057:bool)
                      n1020 = Wait (ms)(milliseconds to wait=u32 100) -> ()  [unwired: 1 out]
                      n1021 = Not(x=w5057) -> (.not. x?=w5055:bool)
                      n1022 = Not(x=w5059) -> (.not. x?=w5058:bool)
                      n1023 = And(x=w5058, y=w5055) -> (x .and. y?=w5056:bool)
                    }
                  }
                  frame #9 {
                    n1024 = property on="Trap Delta (MHz)" class="DigNum (strict)"("Val(Sgnl)"=w5063) -> ()  [unwired: 2 in, 2 out]
                    n1025 = property on="Saved AOD Raster Scan Parameter Sets" class="Arr (strict)"("Index Values"=u32[] [0]) -> ()  [unwired: 2 in, 2 out]
                    n1026 = property on="Save ave N" class="DigNum (strict)"("Val(Sgnl)"=w5061) -> ()  [unwired: 2 in, 2 out]
                  }
                  frame #10 {
                    n1027 = Wait (ms)(milliseconds to wait=u32 500) -> ()  [unwired: 1 out]
                  }
                  frame #11 {
                    n1028 = property on="Load parameters" class="Bool (strict)"("Val(Sgnl)"=TRUE ("Value (Signaling)")) -> ()  [unwired: 2 in, 2 out]
                  }
                }
              }
            }
          }
          frame #7 {
            n1029 = property on="Read Cal" class="Bool (strict)"("Val(Sgnl)"=TRUE ("Value (Signaling)")) -> ()  [unwired: 2 in, 2 out]
          }
          frame #8 {
            n1030 = Wait (ms)(milliseconds to wait=u32 500) -> ()  [unwired: 1 out]
          }
          frame #9 {
            n1031 = property on="Fish for Tether" class="Bool (strict)"("Val(Sgnl)"=FALSE ("Value (Signaling)")) -> ()  [unwired: 2 in, 2 out]
          }
        }
      }
      event "Dump Beads": Value Change {
        # "SCRIPT TO REMOVE BOTH BEADS FROM THE TRAPS. TURNS ON LIGHT WHICH INDICATES THAT STAGE IS MOVING. THEN STOPS SAVING DATA. \nSETS Sample Channel Flow TO TRUE. STOPS INTERLACING GREEN FLUORESCENCE. TURNS OFF Tether INDICATOR BECAUSE WE ARE THROWING IT\nAWAY. SHUTS OFF TRAP POSITION FEEDBACK."
        n1032 = event-data() -> ()  [unwired: 1 in, 5 out]
        n1033 = flat-sequence {
          frame #0 {
            w5070 = FALSE ("Fl. Triggered...")
            w5071 = TRUE ("Stage Moving")
            n1034 = local read "Saving..."() -> (w5072:bool)
            n1035 = local write "Fl. Triggered..."(w5070) -> ()
            n1036 = local write "Stage Moving"(w5071) -> ()
            n1037 = local write "Tether"(w5070) -> ()
            n1038 = property on="Green Laser ON/Interlacing" class="Bool (strict)"("Val(Sgnl)"=w5070) -> ()  [unwired: 2 in, 2 out]
            n1039 = property on="Trap Pos. FB ON" class="Bool (strict)"("Val(Sgnl)"=w5070) -> ()  [unwired: 2 in, 2 out]
            n1040 = property on="Sample Channel Flow" class="Bool (strict)"("Val(Sgnl)"=w5071) -> ()  [unwired: 2 in, 2 out]
            n1041 = local write "Stop Saving"(w5072) -> ()
          }
          frame #1 {
            w5073 = FALSE ("Value (Signaling)")
            # "TURNS TRAPS OFF SO THAT\nBEADS REMAIN AT DUMP \nBEADS POSITION"
            n1042 = property on="Trap 1 (ON/OFF)" class="Bool (strict)"("Val(Sgnl)"=w5073) -> ()  [unwired: 2 in, 2 out]
            n1043 = property on="Trap 2 (ON/OFF)" class="Bool (strict)"("Val(Sgnl)"=w5073) -> ()  [unwired: 2 in, 2 out]
            n1044 = call <vilib>:"Beep.vi"() -> ()  [unwired: 3 in, 9 out]
          }
          frame #2 {
            n1045 = local read "Cal @ (MHz)"() -> (w5074:dbl)
            n1046 = property on="Trap Delta (MHz)" class="DigNum (strict)"("Val(Sgnl)"=w5074) -> ()  [unwired: 2 in, 2 out]
          }
        }
      }
      event "Dip for Protein": Value Change {
        n1047 = event-data() -> ()  [unwired: 1 in, 5 out]
        n1048 = flat-sequence {
          frame #0 {
            n1049 = case shown="True" "Move Trap Before?" {
              frame False {
              }
              frame True {
                n1050 = property on="Trap Delta (MHz)" class="DigNum (strict)"("Val(Sgnl)"="Dip Trap Delta 1 (MHz)") -> ()  [unwired: 2 in, 2 out]
              }
            }
          }
          frame #1 {
            n1051 = Multiply(x="Duration (s)", y=1000.0) -> (x*y=w5078:dbl)
            n1052 = Wait (ms)(milliseconds to wait=w5078) -> ()  [unwired: 1 out]
          }
          frame #2 {
            n1053 = case shown="True" "Move Trap After?" {
              frame False {
              }
              frame True {
                n1054 = property on="Trap Delta (MHz)" class="DigNum (strict)"("Val(Sgnl)"="Dip Trap Delta 2 (MHz)") -> ()  [unwired: 2 in, 2 out]
              }
            }
          }
          frame #3 {
            n1055 = case shown="True" "Green ON After?" {
              frame False {
              }
              frame True {
                n1056 = property on="Green Laser ON/Interlacing" class="Bool (strict)"("Val(Sgnl)"=TRUE ("Value (Signaling)")) -> ()  [unwired: 2 in, 2 out]
              }
            }
          }
          frame #4 {
            n1057 = Wait (ms)(milliseconds to wait=u32 500) -> ()  [unwired: 1 out]
          }
          frame #5 {
            n1058 = case shown="True" "Save Data After?" {
              frame False {
              }
              frame True {
                n1059 = property on="Start Saving" class="Bool (strict)"("Val(Sgnl)"=TRUE ("Value (Signaling)")) -> ()  [unwired: 2 in, 2 out]
              }
            }
          }
        }
      }
      event "Profile": Value Change {
        n1060 = event-data() -> ()  [unwired: 1 in, 5 out]
        n1061 = flat-sequence {
          frame #0 {
            w5088 = 0.0 ("element")
            n1062 = Build Array(w5088, "Y change (mm)", w5088) -> ()  [unwired: 1 out]
          }
          frame #1 {
            # "stop saving"
            n1063 = local write "Stop Saving"(TRUE ("Stop Saving")) -> ()
            n1064 = local write "Stage Moving"(FALSE ("Stage Moving")) -> ()
          }
        }
      }
      event "Got ADig bead": Value Change {
        n1065 = event-data() -> ()  [unwired: 1 in, 5 out]
        n1066 = property on="Move Cap. 1 (DNA Top)" class="Bool (strict)"("Val(Sgnl)"=TRUE ("Value (Signaling)")) -> ()  [unwired: 2 in, 2 out]
        n1067 = property on="Inject Bottom" class="Bool (strict)"("Val(Sgnl)"=FALSE ("Value (Signaling)")) -> ()  [unwired: 2 in, 2 out]
      }
      event "Got DNA bead": Value Change {
        n1068 = event-data() -> ()  [unwired: 1 in, 5 out]
        n1069 = property on="Cal/Data Acq. Spot" class="Bool (strict)"("Val(Sgnl)"=TRUE ("Value (Signaling)")) -> ()  [unwired: 2 in, 2 out]
        n1070 = property on="Inject Top" class="Bool (strict)"("Val(Sgnl)"=FALSE ("Value (Signaling)")) -> ()  [unwired: 2 in, 2 out]
      }
      event "Take Stepping Data": Value Change {
        n1071 = event-data() -> ()  [unwired: 1 in, 5 out]
        n1072 = local read "Save ave N"() -> (w5106:dbl)
        n1073 = flat-sequence {
          tunnel: w5106 -> [w5108]
          tunnel: [w5108] -> w5101
          tunnel: [w5110] -> w5102
          tunnel: w5101 -> [w5110]
          tunnel: [w5112] -> w5103
          tunnel: w5102 -> [w5112]
          tunnel: [w5115] -> w5104
          tunnel: w5103 -> [w5115]
          tunnel: [w5117] -> w5105
          tunnel: w5104 -> [w5117]
          tunnel: [w5119] -> w5099
          tunnel: w5105 -> [w5119]
          tunnel: w5099 -> [w5122]
          tunnel: [w5122] -> w5098
          tunnel: w5098 -> [w5123]
          tunnel: [w5123] -> w5100
          tunnel: w5100 -> [w5129]
          frame #0 {
            n1074 = property on="Save ave N" class="DigNum (strict)"("Val(Sgnl)"="Save ave factor") -> ()  [unwired: 2 in, 2 out]
          }
          frame #1 {
            n1075 = Wait (ms)(milliseconds to wait=u32 100) -> ()  [unwired: 1 out]
          }
          frame #2 {
            n1076 = local read "Offset 2 Start (MHz)"() -> (w5114:dbl)
            n1077 = property on="Saved AOD Raster Scan Parameter Sets" class="Arr (strict)"("Index Values"=u32[] [2]) -> ()  [unwired: 2 in, 2 out]
            n1078 = property on="Trap Delta (MHz)" class="DigNum (strict)"("Val(Sgnl)"=w5114) -> ()  [unwired: 2 in, 2 out]
          }
          frame #3 {
            n1079 = property on="Load parameters" class="Bool (strict)"("Val(Sgnl)"=TRUE ("Value (Signaling)")) -> ()  [unwired: 2 in, 2 out]
          }
          frame #4 {
            n1080 = Wait (ms)(milliseconds to wait=u32 100) -> ()  [unwired: 1 out]
          }
          frame #5 {
            n1081 = property on="Trap Raster Scan" class="Bool (strict)"("Val(Sgnl)"=TRUE ("Value (Signaling)")) -> ()  [unwired: 2 in, 2 out]
          }
          frame #6 {
            n1082 = Wait (ms)(milliseconds to wait=u32 1000) -> ()  [unwired: 1 out]
          }
          frame #7 {
            n1083 = while {
              stop <- w5126 stop-if-true
              n1084 = local read "Raster Scanning..."() -> (w5128:bool)
              n1085 = local read "Saving..."() -> (w5127:bool)
              n1086 = Not(x=w5127) -> (.not. x?=w5124:bool)
              n1087 = Not(x=w5128) -> (.not. x?=w5125:bool)
              n1088 = And(x=w5125, y=w5124) -> (x .and. y?=w5126:bool)
            }
          }
          frame #8 {
            n1089 = property on="Save ave N" class="DigNum (strict)"("Val(Sgnl)"=w5129) -> ()  [unwired: 2 in, 2 out]
          }
        }
      }
      event "Step Size (nm)": Value Change {
        n1090 = event-data() -> ()  [unwired: 1 in, 5 out]
        n1091 = flat-sequence {
          frame #0 {
            n1092 = property on="Saved AOD Raster Scan Parameter Sets" class="Arr (strict)"("Index Values"=u32[] [1]) -> ()  [unwired: 2 in, 2 out]
          }
          frame #1 {
            n1093 = Multiply(x="N Steps", y="Step Size (nm)") -> (x*y=w5131:dbl)
            n1094 = property on="Scan Speed AOD (nm/s) 2" class="DigNum (strict)"("Value"="Step Size (nm)") -> ()  [unwired: 2 in, 2 out]
            n1095 = property on="Step Size AOD (nm) 2" class="DigNum (strict)"("Value"="Step Size (nm)") -> ()  [unwired: 2 in, 2 out]
            n1096 = property on="Scan Range AOD (nm) 2" class="DigNum (strict)"("Value"=w5131) -> ()  [unwired: 2 in, 2 out]
          }
        }
      }
      event "Take Detection Laser\nImage": Value Change {
        n1097 = event-data() -> ()  [unwired: 1 in, 5 out]
        n1098 = flat-sequence {
          tunnel: [w5159] -> w5149
          tunnel: [w5158] -> w5142
          tunnel: [w5157] -> w5134
          tunnel: [w5162] -> w5150
          tunnel: w5149 -> [w5162]
          tunnel: [w5161] -> w5143
          tunnel: w5142 -> [w5161]
          tunnel: [w5160] -> w5135
          tunnel: w5134 -> [w5160]
          tunnel: [w5166] -> w5151
          tunnel: w5150 -> [w5166]
          tunnel: [w5165] -> w5144
          tunnel: w5143 -> [w5165]
          tunnel: [w5164] -> w5136
          tunnel: w5135 -> [w5164]
          tunnel: [w5172] -> w5152
          tunnel: w5151 -> [w5172]
          tunnel: [w5171] -> w5145
          tunnel: w5144 -> [w5171]
          tunnel: [w5170] -> w5137
          tunnel: w5136 -> [w5170]
          tunnel: [w5176] -> w5153
          tunnel: w5152 -> [w5176]
          tunnel: [w5175] -> w5146
          tunnel: w5145 -> [w5175]
          tunnel: [w5174] -> w5138
          tunnel: w5137 -> [w5174]